vi "Visualizacion_NEW.vi"() -> ()   [LabVIEW 2021]
uses:
  <vilib>/Modbus/master/Modbus Master.lvclass
  <vilib>/Modbus/master/Create Master Instance (TCP).vi
panel:
  out "LEL":bool
  out "CO":bool
  out "O2":bool
  out "Contador Ciclos":sgl
  out "LEL":sgl
  out "CO":sgl
  out "O2":sgl
  in  "SP Temperatura (CC)":dbl=25.0 min=-42.0 max=55.0
  in  "SP HR (CC)":dbl=10.0
  out "DI Sim Bitron Param":bool
  out "Parameters":u16[](array[numeric])
  out "Error":bool
  out "Warning":bool
  out "MEAN (T)":sgl format="%0.2f"
  out "Peltiers enable":bool
  out "Program Status":bool
  out "SP (T)":sgl
  out "Segmento_temp":u16
  in  "?":T1(tab)
  in  "?":T2(tab)
  out "TEMPERATURA MEDIA":dynamicdata(graph)
  out "ALL TOGETHER":dynamicdata(graph)
  out "VALVULA 1  BOBINAS 1 Y 2":dynamicdata(graph)
  out "VALVULA 2 Y BOBINA 3 Y 4":dynamicdata(graph)
  out "VALVULA 3 Y BOBINA 5 Y 6":dynamicdata(graph)
  out "VALVULA 4 Y BOBINA 7 Y 8":dynamicdata(graph)
  out "O2/CO/LEL":dynamicdata(graph)
  out "Camara climatica":dynamicdata(graph)
  out "current time":timestamp
  out "W1.16":bool
  out "W1.15":bool
  out "W1.11":bool
  out "W1.10":bool
  out "W1.14":bool
  out "W1.13":bool
  out "W1.12":bool
  out "W1.1":bool
  out "W2":bool
  out "W3":bool
  out "W4":bool
  out "W1.2":bool
  out "W1.3":bool
  out "W1.6":bool
  out "W1.5":bool
  out "W1.4":bool
  out "W1.9":bool
  out "W1.8":bool
  out "W1.7":bool
  out "warnings table":T3(array[cluster]) {"Time Stamp" format="%<%.3X %x>T"}
  in  "Reset":bool
  out "Comunicacion Modbus":errorcluster
  in  "trigger bob frio (ºC)":dbl=-27.5 min=-40.0 max=80.0
  in  "Offset de ciclo.":dbl min=-40.0 max=80.0
  in  "Digital Input Bitron Simulation":bool
  in  "Pelt ºC/min":dbl=6.0
  in  "Cam ºC/min":dbl=100.0
  in  "Tiempo máximo de ciclo(min)":dbl=140.0
  in  "Setpoint corte frío(ºC)":dbl=-30.0 min=-42.0 max=80.0
  in  "Setpoint Frío(ºC)":dbl=-33.0 min=-42.0 max=80.0
  in  "Setpoint peltiers(ºC)":dbl=85.0 min=-42.0 max=80.0
  in  "Tiempo estabilidad de Frío(min)":dbl=15.0
  in  "Tiempo mínimo de ciclo(min)":dbl=70.0
  in  "Setpoint calor corte rampa(ºC)":dbl=51.0 min=-40.0 max=80.0
  in  "Tiempo ciclo (Bitron FSM Sim)":dbl=95.0
  in  "Setpoint calor cam":dbl=55.0 min=-40.0 max=80.0
  in  "Tiempo Ciclo 0 (min)":dbl=5.0
  in  "Save Parameters":bool
  out "Ventil 2":sgl
  out "Ventil 3":sgl format="%#.2g"
  out "Temp bob 1 (P)":sgl format="%#.2g"
  out "Temp bob 3 (P)":sgl
  out "Ventil 4":sgl
  out "Ventil 1":sgl format="%#.2g"
  out "Temp Bob 5 (P)":sgl format="%#.2g"
  in  "PWM 4(SP)":u16
  in  "PWM 3(SP) 2":u16
  in  "PWM 2(SP) 2":u16
  in  "PWM 1(SP) 2":u16
  in  "Test PWM (%)":bool
  in  "Conf PIDs":bool
  in  "TestPID 4(ºC)":u16
  in  "TestPID3(ºC)":u16
  in  "TestPID 2(ºC)":u16
  in  "TestPID 1(ºC)":u16
  out "Temp Man 2":sgl
  out "PWM 1(SP)":u16
  out "Temp Man 3":sgl format="%#.2g"
  out "Temp Man 1":sgl format="%#.2g"
  out "Temp Man 4":sgl
  out "PWM 2(SP)":u16
  out "PWM 3(SP)":u16
  out "PWM 4(SP)":u16
  out "Temp bob 7 (P)":sgl
  out "Temp bob 2 (Sh)":sgl
  out "Temp bob  4 (Sh)":sgl
  out "Temp bob 6 (Sh)":sgl format="%#.2g"
  out "Temp bob 8 (Sh)":sgl
  in  "Descarte Media Temps":u16 max=3 step=1
  in  "Enable PI 1":bool=TRUE
  in  "Enable PI 2":bool=TRUE
  in  "Enable PI 3":bool=TRUE
  in  "Enable PI 4":bool=TRUE
  in  "Test PID (ºC)":bool
  out "DISK":sgl(graph)
  out "RAM":sgl(graph)
  in  "Tiempo de guardado":u32=600
  out "data to be saved":dbl[][](array[numeric])
  out "Guardando en disco":bool
  out "array w/ subset deleted":dbl[][](array[numeric])
  out "size(s)":i32
  out "W to save":string[][](array[string])
  in  "Warning saved":bool
  in  "Tiempo/dato (s)":u32=1
  out "USO DE DISCO(%)":sgl
  out "USO DE RAM (%)":sgl
  out "DO H2 Lab":bool
  in  "Guardar datos":bool=TRUE
  out "senal_bitron":bool
  in  "Stop Ensayo":bool
  out "Coils write":bool[](array[boolean])
  out "Int values":u16[](array[numeric])
  out "SGL values":sgl[](array[numeric])
  out "coil values":bool[](array[boolean])
  out "ComunicacionCRIO":bool
  in  "run_program":bool
  out "Setpoint_temp_write":dbl
  out "Setpoint_hum_write":dbl
  out "Temperatura Camara":dbl
  out "Humedad relativa (HR)":dbl
  in  "Pause_Entrar_camara":bool
  in  "Pause":bool
  in  "stop":bool
  in  "Tab Control":T4(tab)
  out "T Man 4":dbl(slide) scale=-45.0..100.0
  out "T Man 3":dbl(slide) scale=-45.0..100.0
  out "T Man 2":dbl(slide) scale=-45.0..100.0
  out "T Man 1":dbl(slide) scale=-45.0..100.0
  out "T Bob 1":dbl(slide) scale=-40.0..95.0
  out "T Bob 3":dbl(slide) scale=-40.0..95.0
  out "T Bob 5":dbl(slide) scale=-40.0..100.0
  out "T bob 9":dbl(slide) scale=-40.0..95.0
  out "T bob 10":dbl(slide) scale=-40.0..95.0
  out "T bob 11":dbl(slide) scale=-40.0..95.0
  out "T Bob 7":dbl(slide) scale=-40.0..95.0
  out "T bob 12":dbl(slide) scale=-45.0..95.0
  out "T bob 8":dbl(slide) scale=-45.0..95.0
  out "T bob 7":dbl(slide) scale=-45.0..95.0
  out "T bob 6":dbl(slide) scale=-45.0..95.0
  out "Ventil 5":dbl(slide) scale=-45.0..95.0
  # "Control Programa Principal"
  # "Control Manual CC"
  # "%"
  # "ºC"
  # "Cámara climática"
  # "ºC"
  # "ºC"
  # "%"
  # "%"
  # "Simulación señal Bitron"
  # "ºC"
  # "HR"
  # "TempCC"
  # "SP_HR"
  # "SP_TempCC"
  # "Mean T"
  # "Warnings y Errores"
  # "Warning Valvulas"
  # "Warning Bobinas"
  # "Parametros y configuracion para la curva de ciclado"
  # "ºC"
  # "VALVE 4"
  # "ºC"
  # "ºC"
  # "Fan Right"
  # "%"
  # "ºC"
  # "ºC"
  # "VALVE 3"
  # "ºC"
  # "ºC"
  # "%"
  # "Fan Mid-Right"
  # "ºC"
  # "ºC"
  # "VALVE 2"
  # "ºC"
  # "ºC"
  # "%"
  # "Fan Mid-Left"
  # "ºC"
  # "ºC"
  # "VALVE 1"
  # "ºC"
  # "ºC"
  # "%"
  # "Fan Left"
  # "ºC"
  # "ºC"
  # "1 Dato\n----------------"
  # "Frecuencia de guardado:"
  # "s"
  # "s"
  # "T Manifolds:"
  # "1                              2                                 3                                  4"
  # "T Bobinas:"
  # "1               2               3               4               5                 6               7               8"
  # "V1"
  # "V2"
  # "V3"
  # "V4"
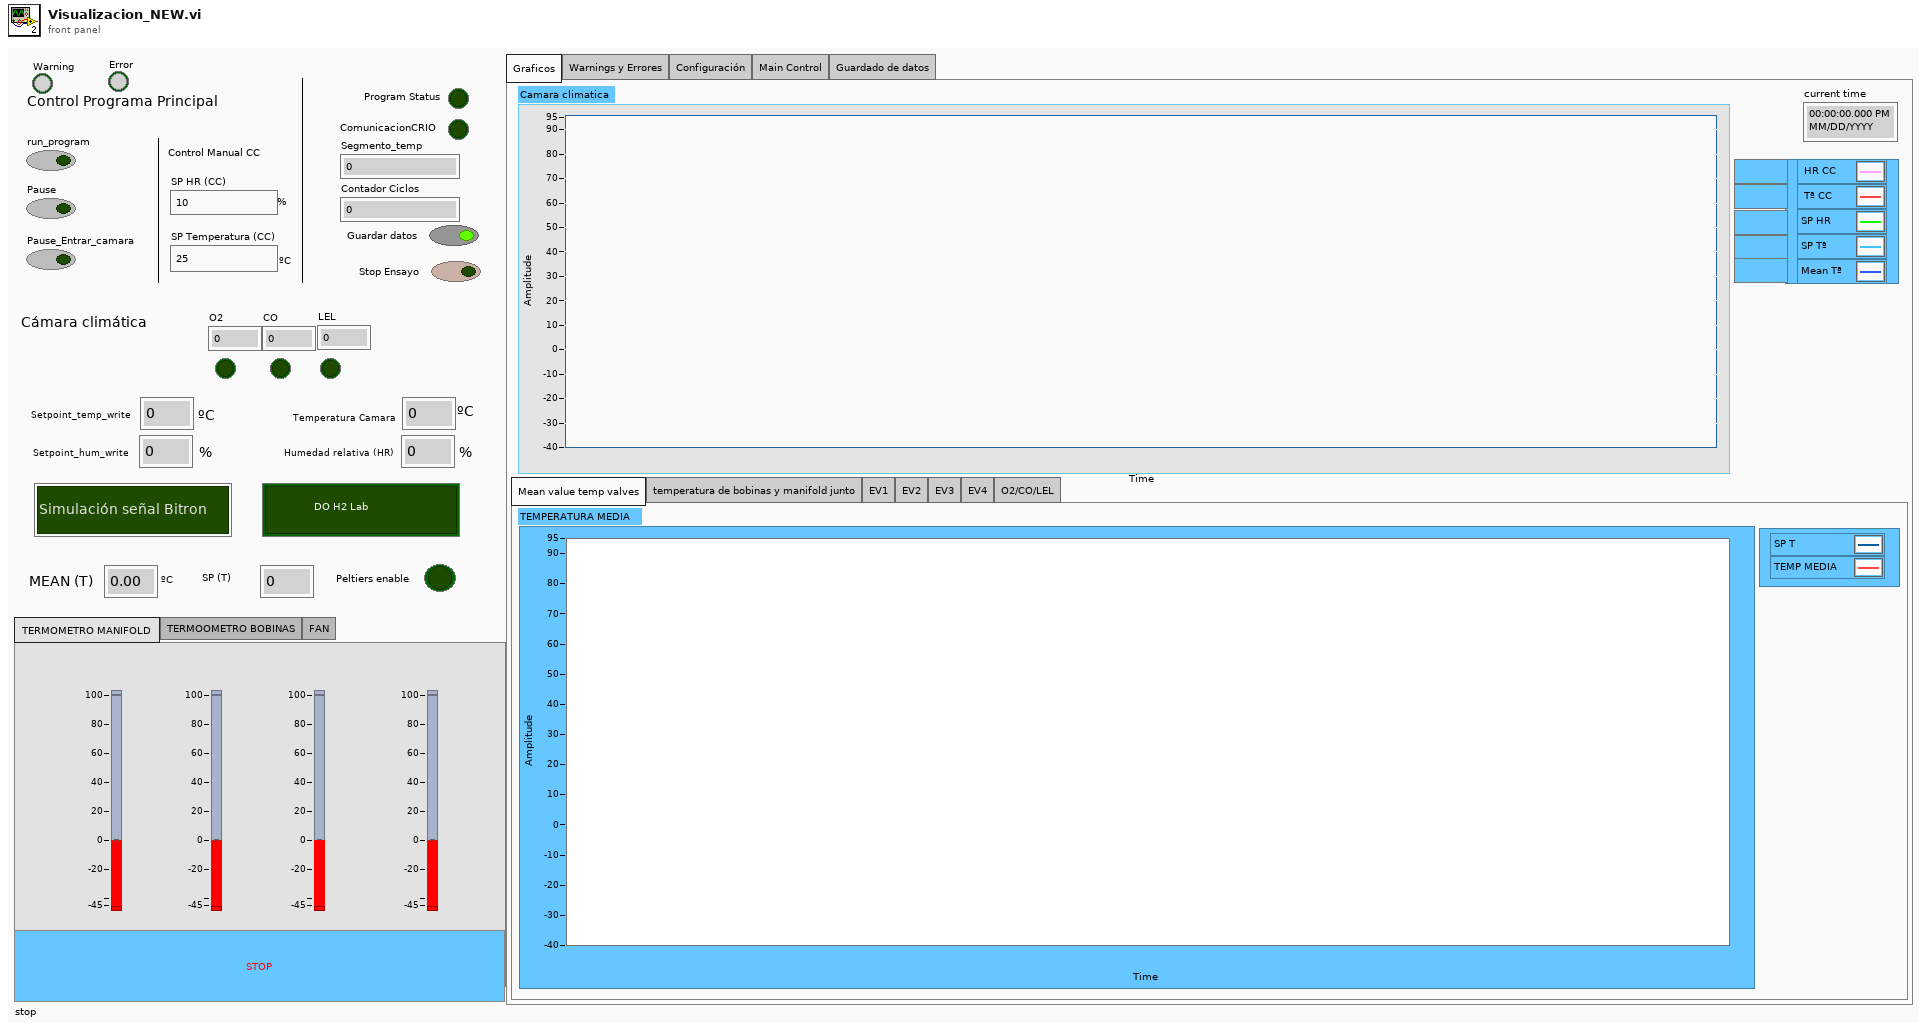
[diagram p1: front panel]
types:
  T1 = enum32{"Graficos", "Warnings y Errores", "Configuración", "Main Control", "Guardado de datos"}
  T2 = enum32{"Mean value temp valves", "temperatura de bobinas y manifold junto", "EV1", "EV2", "EV3", "EV4", "O2/CO/LEL"}
  T3 = cluster{"Time Stamp":timestamp, "Descripcion":string, "Numeric":i32}[]
  T4 = enum32{"TERMOMETRO MANIFOLD ", "TERMOOMETRO BOBINAS", "FAN"}
  T5 = enum8{"Enabled", "Disabled", "Disabled and Grayed Out"}
  T6 = enum16{"open", "open or create", "create or replace", "create", "open (read-only)"}
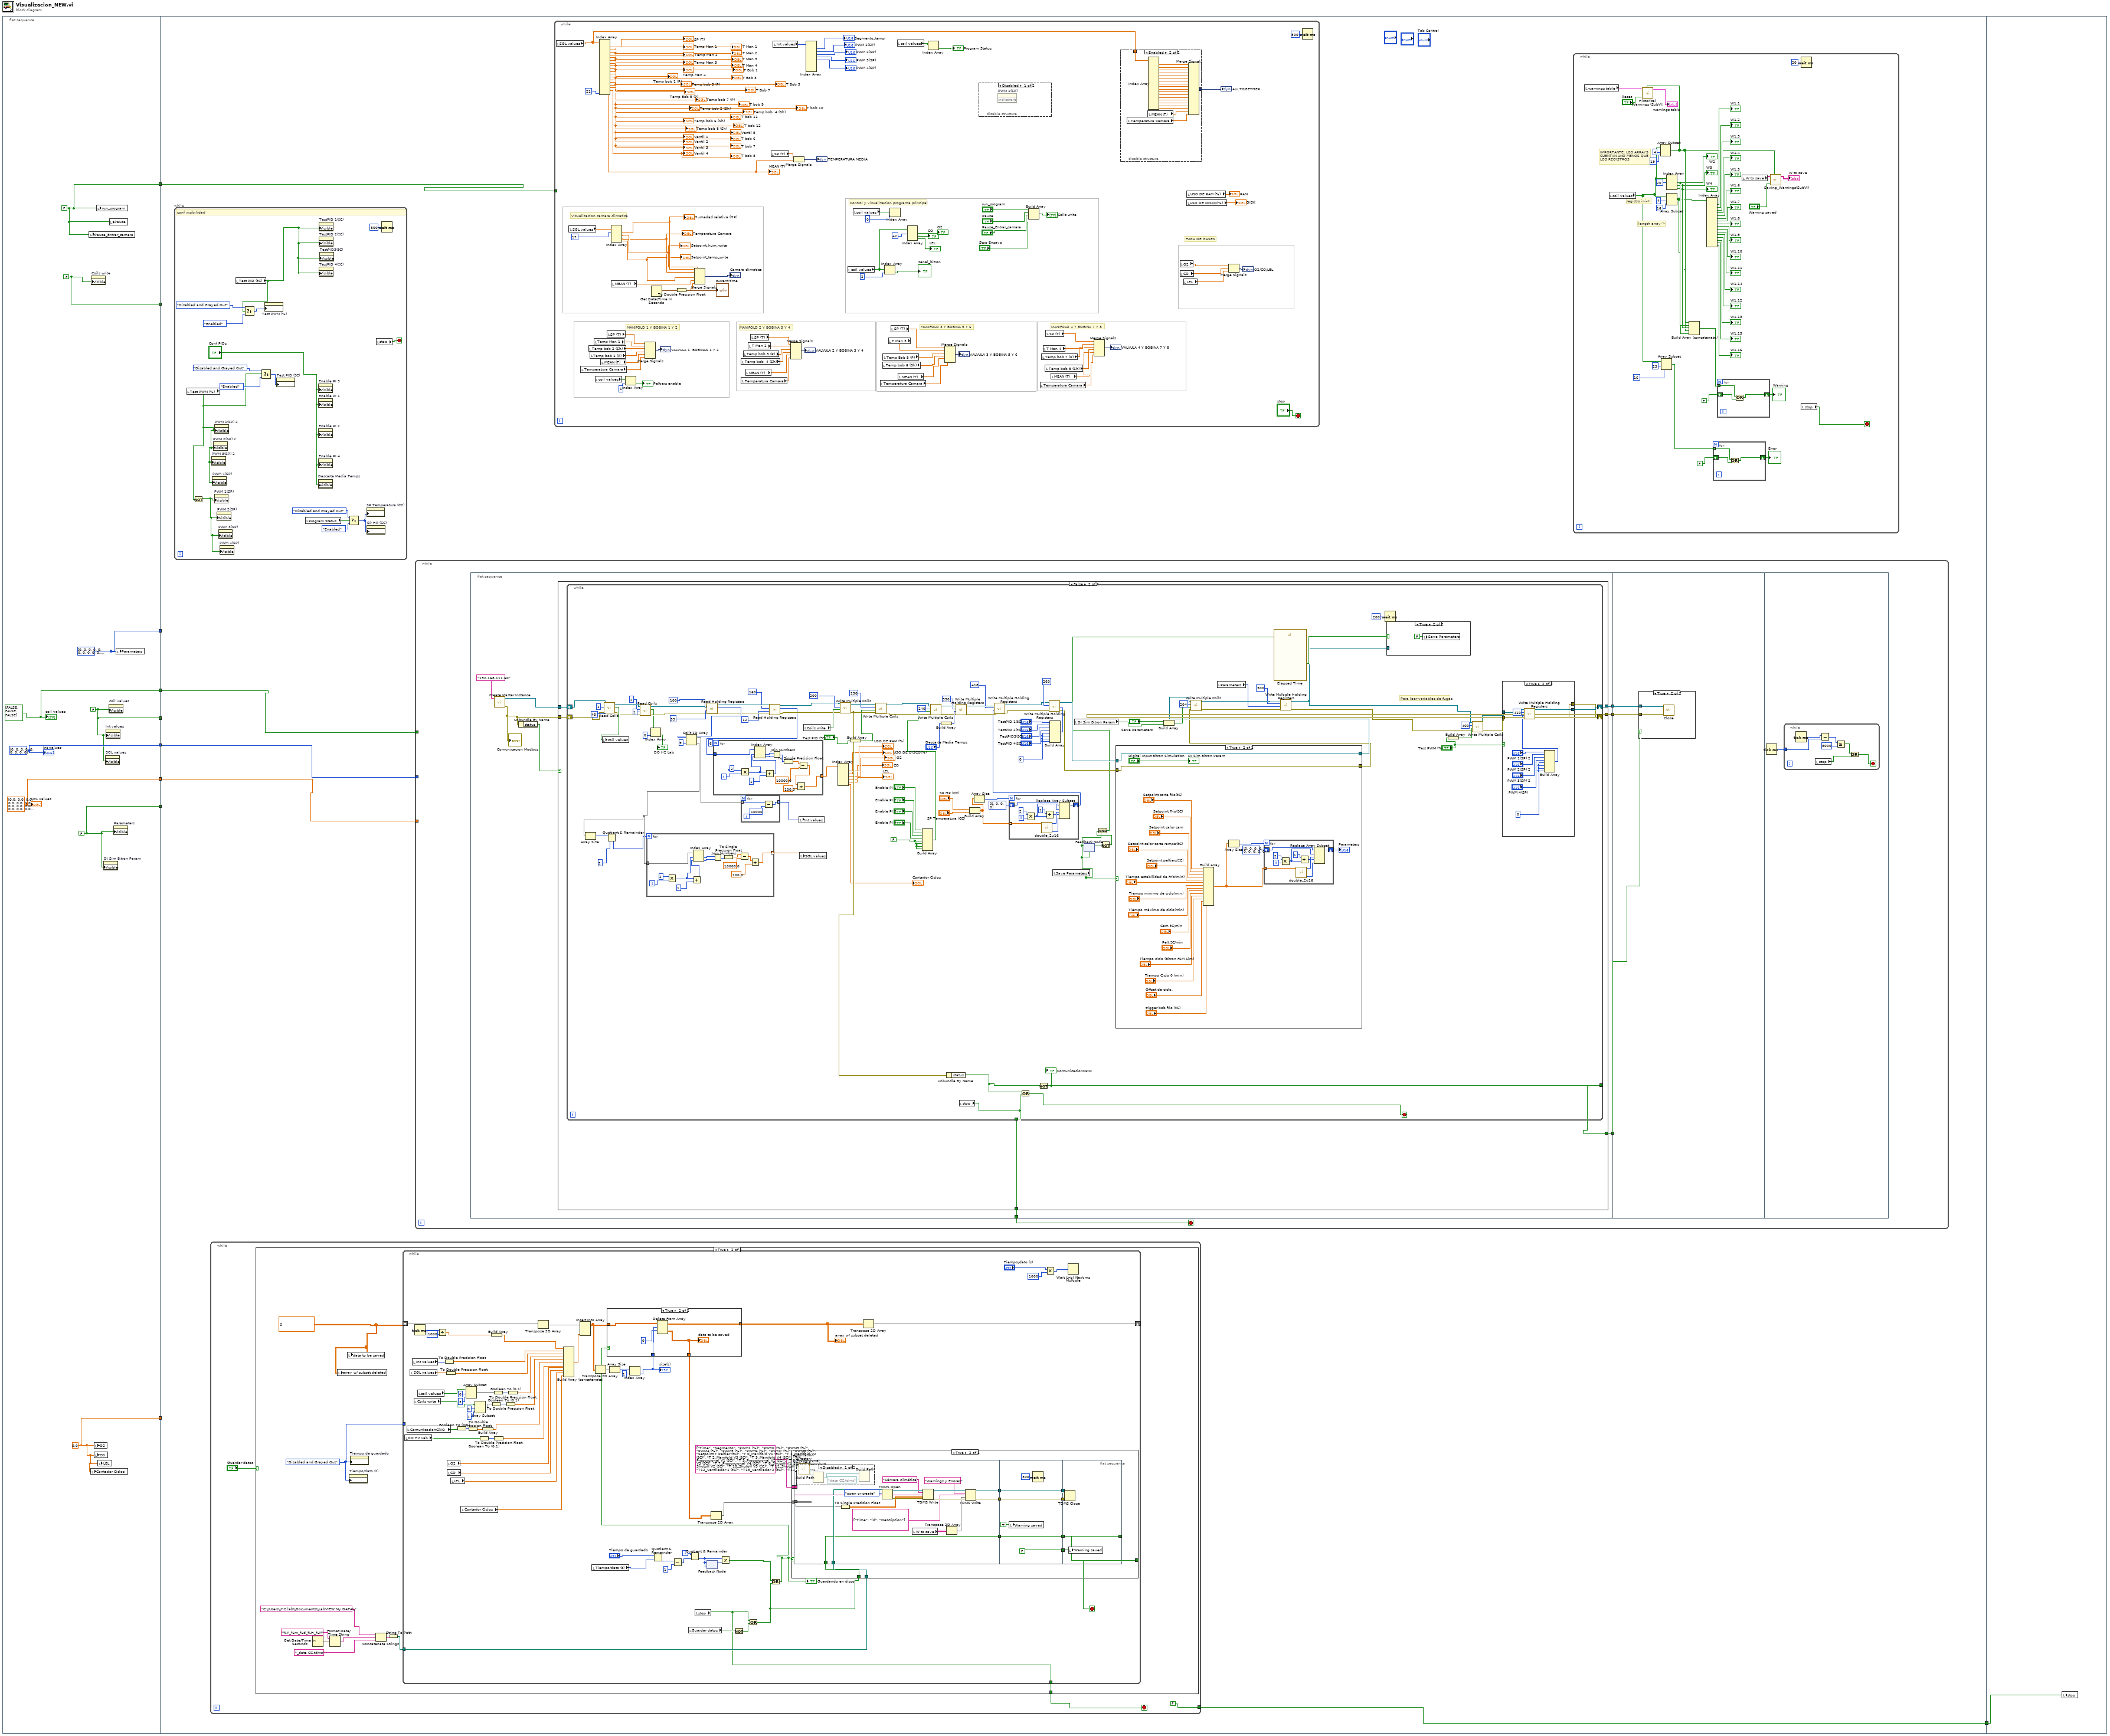
[diagram p0: block diagram]
diagram:
  n1 = flat-sequence {
    tunnel: [w19] -> w10
    tunnel: [w18] -> w9
    tunnel: [w17] -> w8
    tunnel: [w16] -> w7
    tunnel: [w14] -> w5
    tunnel: [w15] -> w4
    tunnel: [w13] -> w3
    tunnel: [w12] -> w2
    tunnel: [w11] -> w1
    tunnel: w10 -> [w24]
    tunnel: w9 -> [w23]
    tunnel: w8 -> [w22]
    tunnel: w7 -> [w21]
    tunnel: [w20] -> w6
    tunnel: w5 -> [_]
    tunnel: w4 -> [_]
    tunnel: w3 -> [_]
    tunnel: w2 -> [_]
    tunnel: w1 -> [_]
    tunnel: w6 -> [w583]
    frame #0 {
      w11 = sgl 0.0 ("O2")
      w12 = u16[] [0, 0, 0, 0, 0, 0, 0, 0, 0, 0, 0, 0, 0, 0, 0, 0, 0, 0, 0, 0, 0, 0] ("Parameters")
      w13 = FALSE ("Visible")
      w15 = FALSE ("Visible")
      w14 = FALSE ("Visible")
      w17 = sgl[] [0.0, 0.0, 0.0, 0.0, 0.0, 0.0, 0.0, 0.0, 0.0, 0.0, 0.0, 0.0, 0.0, 0.0, 0.0, 0.0, 0.0, 0.0, 0.0, 0.0, 0.0, 0.0] ("SGL values")
      w18 = u16[] [0, 0, 0, 0, 0, 0, 0, 0, 0] ("Int values")
      w16 = FALSE ("run_program")
      w19 = bool[] [FALSE, FALSE, FALSE] ("coil values")
      n2 = local write "Pause_Entrar_camara"(w16) -> ()
      n3 = local write "Contador Ciclos"(w11) -> ()
      n4 = property on="Coils write" class="Arr (strict)"("Visible"=w15) -> ()  [unwired: 2 in, 2 out]
      n5 = local write "O2"(w11) -> ()
      n6 = local write "CO"(w11) -> ()
      n7 = local write "run_program"(w16) -> ()
      n8 = local write "LEL"(w11) -> ()
      n9 = property on="DI Sim Bitron Param" class="Bool (strict)"("Visible"=w13) -> ()  [unwired: 2 in, 2 out]
      n10 = property on="SGL values" class="Arr (strict)"("Visible"=w14) -> ()  [unwired: 2 in, 2 out]
      n11 = property on="Int values" class="Arr (strict)"("Visible"=w14) -> ()  [unwired: 2 in, 2 out]
      n12 = property on="coil values" class="Arr (strict)"("Visible"=w14) -> ()  [unwired: 2 in, 2 out]
      n13 = local write "Pause"(w16) -> ()
      n14 = property on="Parameters" class="Arr (strict)"("Visible"=w13) -> ()  [unwired: 2 in, 2 out]
      n15 = local write "Parameters"(w12) -> ()
      "coil values" <- w19
      "Int values" <- w18
      "SGL values" <- w17
    }
    frame #1 {
      n16 = while {
        stop <- w40 stop-if-true
        # "conf visibilidad"
        n17 = local read "Test PWM (%)"() -> (w29:bool)
        n18 = Not(x=w29) -> (.not. x?=w37:bool)
        n19 = property on="PWM 3(SP) 2" class="DigNum (strict)"("Visible"=w29) -> ()  [unwired: 2 in, 2 out]
        n20 = property on="PWM 4(SP)" class="DigNum (strict)"("Visible"=w29) -> ()  [unwired: 2 in, 2 out]
        n21 = property on="PWM 2(SP) 2" class="DigNum (strict)"("Visible"=w29) -> ()  [unwired: 2 in, 2 out]
        n22 = property on="PWM 1(SP)" class="DigNum (strict)"("Visible"=w37) -> ()  [unwired: 2 in, 2 out]
        n23 = property on="PWM 1(SP) 2" class="DigNum (strict)"("Visible"=w29) -> ()  [unwired: 2 in, 2 out]
        n24 = property on="PWM 2(SP)" class="DigNum (strict)"("Visible"=w37) -> ()  [unwired: 2 in, 2 out]
        n25 = property on="PWM 3(SP)" class="DigNum (strict)"("Visible"=w37) -> ()  [unwired: 2 in, 2 out]
        n26 = property on="PWM 4(SP)" class="DigNum (strict)"("Visible"=w37) -> ()  [unwired: 2 in, 2 out]
        n27 = local read "Test PID (ºC)"() -> (w33:bool)
        n28 = Select(t=T5."Disabled and Grayed Out" ("Disabled"), s=w33, f=T5."Enabled" ("Disabled")) -> (s? t:f=w34:T5)
        n29 = Select(t=T5."Disabled and Grayed Out" ("Disabled"), s=w29, f=T5."Enabled" ("Disabled")) -> (s? t:f=w30:T5)
        n30 = property on="Test PWM (%)" class="Bool (strict)"("DisabledEnum"=w34) -> ()  [unwired: 2 in, 2 out]
        n31 = property on="Test PID (ºC)" class="Bool (strict)"("DisabledEnum"=w30) -> ()  [unwired: 2 in, 2 out]
        n32 = local read "Program Status"() -> (w28:bool)
        n33 = property on="Descarte Media Temps" class="DigNum (strict)"("Visible"="Conf PIDs") -> ()  [unwired: 2 in, 2 out]
        n34 = property on="Enable PI 3" class="Bool (strict)"("Visible"="Conf PIDs") -> ()  [unwired: 2 in, 2 out]
        n35 = property on="Enable PI 1" class="Bool (strict)"("Visible"="Conf PIDs") -> ()  [unwired: 2 in, 2 out]
        n36 = property on="Enable PI 2" class="Bool (strict)"("Visible"="Conf PIDs") -> ()  [unwired: 2 in, 2 out]
        n37 = property on="Enable PI 4" class="Bool (strict)"("Visible"="Conf PIDs") -> ()  [unwired: 2 in, 2 out]
        n38 = property on="TestPID 1(ºC)" class="DigNum (strict)"("Visible"=w33) -> ()  [unwired: 2 in, 2 out]
        n39 = property on="TestPID 2(ºC)" class="DigNum (strict)"("Visible"=w33) -> ()  [unwired: 2 in, 2 out]
        n40 = property on="TestPID 4(ºC)" class="DigNum (strict)"("Visible"=w33) -> ()  [unwired: 2 in, 2 out]
        n41 = property on="TestPID3(ºC)" class="DigNum (strict)"("Visible"=w33) -> ()  [unwired: 2 in, 2 out]
        n42 = Select(t=T5."Disabled and Grayed Out" ("Disabled"), s=w28, f=T5."Enabled" ("Disabled")) -> (s? t:f=w25:T5)
        n43 = property on="SP Temperatura (CC)" class="DigNum (strict)"("DisabledEnum"=w25) -> ()  [unwired: 2 in, 2 out]
        n44 = property on="SP HR (CC)" class="DigNum (strict)"("DisabledEnum"=w25) -> ()  [unwired: 2 in, 2 out]
        n45 = local read "stop"() -> (w40:bool)
        n46 = Wait (ms)(milliseconds to wait=u32 500) -> ()  [unwired: 1 out]
      }
      n47 = while {
        tunnel: [FALSE ("stop Control General")] -> w20
        stop <- w91 stop-if-true
        n48 = case shown="True" "Guardar datos" {
          tunnel: [w94 w97] -> w91
          frame False {
            w93 = T5."Enabled" ("Disabled")
            n49 = property on="Tiempo/dato (s)" class="DigNum (strict)"("DisabledEnum"=w93) -> ()  [unwired: 2 in, 2 out]
            n50 = property on="Tiempo de guardado" class="DigNum (strict)"("DisabledEnum"=w93) -> ()  [unwired: 2 in, 2 out]
            n51 = local read "stop"() -> (w94:bool)
            n52 = Wait Until Next ms Multiple(millisecond multiple=u32 1000 ("milliseconds to wait")) -> ()  [unwired: 1 out]
          }
          frame True {
            w96 = T5."Disabled and Grayed Out" ("Disabled")
            w105 = dbl[][] []
            n53 = Get Date/Time In Seconds() -> (seconds since 1Jan1904=w104:timestamp)
            n54 = Format Date/Time String(time format string (%c)="%Y_%m_%d_%H_%M", seconds (now)=w104) -> (date/time string=w101:string)  [unwired: 1 in]
            n55 = local write "array w/ subset deleted"(w105) -> ()
            n56 = local write "data to be saved"(w105) -> ()
            n57 = property on="Tiempo/dato (s)" class="DigNum (strict)"("DisabledEnum"=w96) -> ()  [unwired: 2 in, 2 out]
            n58 = property on="Tiempo de guardado" class="DigNum (strict)"("DisabledEnum"=w96) -> ()  [unwired: 2 in, 2 out]
            n59 = Concatenate Strings("C:\\Users\\H2.lab\\Documents\\LabVIEW My DATA\\" ("string"), w101, "_data CC.tdms" ("string")) -> (w102:string)
            n60 = String To Path(string=w102) -> (path=w99:path)
            n61 = while {
              shift-right: [w160] -> _
              shift-left: w105 -> [w163]
              tunnel: w99 -> [w153]
              tunnel: [w131] -> w97
              tunnel: w96 -> [_]
              i -> [w167]
              stop <- w135 stop-if-true
              n62 = local read "DO H2 Lab"() -> (w129:bool)
              n63 = local read "ComunicacionCRIO"() -> (w137:bool)
              n64 = local read "SGL values"() -> (w151:sgl[])
              n65 = local read "Int values"() -> (w152:u16[])
              n66 = local read "Coils write"() -> (w123:bool[])
              n67 = Tick Count (ms)() -> (millisecond timer value=w155:u32)
              n68 = local read "coil values"() -> (w127:bool[])
              n69 = Divide(x=w155, y=u32 1000) -> (x/y=w148:dbl)
              n70 = To Double Precision Float(number=w152) -> (double precision float=w150:dbl[])
              n71 = To Double Precision Float(number=w151) -> (double precision float=w149:dbl[])
              n72 = local read "O2"() -> (w110:sgl)
              n73 = local read "CO"() -> (w109:sgl)
              n74 = local read "LEL"() -> (w108:sgl)
              n75 = Boolean To (0,1)(Boolean=w137) -> (0, 1=w144:i16)
              n76 = local read "Contador Ciclos"() -> (w107:sgl)
              n77 = Array Subset(array=w127, index=0, length=3) -> (w126:bool[])
              n78 = To Double Precision Float(number=w144) -> (double precision float=w143:dbl)
              n79 = Array Subset(array=w123, index=0, length=4) -> (w120:bool[])
              n80 = Boolean To (0,1)(Boolean=w129) -> (0, 1=w130:i16)
              n81 = Build Array(w143) -> (w140:dbl[])
              n82 = Boolean To (0,1)(Boolean=w120) -> (0, 1=w139:i16[])
              n83 = Build Array(w148) -> (w147:dbl[])
              n84 = Boolean To (0,1)(Boolean=w126) -> (0, 1=w146:i16[])
              n85 = To Double Precision Float(number=w130) -> (double precision float=w128:dbl)
              n86 = To Double Precision Float(number=w139) -> (double precision float=w138:dbl[])
              n87 = To Double Precision Float(number=w146) -> (double precision float=w145:dbl[])
              n88 = Transpose 2D Array(2D array=w163) -> (transposed array=w162:dbl[][])
              n89 = Build Array (concatenate)(w147, w150, w149, w145, w138, w140, w128, w110, w109, w108, w107) -> (w168:dbl[])
              n90 = Insert Into Array(array=w162, new element=w168) -> (w165:dbl[][])  [unwired: 2 in]
              n91 = local read "Tiempo/dato (s)"() -> (w115:u32)
              n92 = Transpose 2D Array(2D array=w165) -> (transposed array=w159:dbl[][])
              n93 = Array Size(array=w159) -> (size(s)=w158:i32[])
              n94 = Index Array(array=w158, index=1) -> (element=w157:i32)
              "size(s)" <- w157
              n95 = Quotient & Remainder(x="Tiempo de guardado", y=w115) -> (floor(x/y)=w114:u32)  [unwired: 1 out]
              n96 = Subtract(x=w114, y=u32 1) -> (x-y=w113:u32)
              n97 = local read "Guardar datos"() -> (w134:bool)
              n98 = Quotient & Remainder(x=w167, y=w113) -> (floor(x/y)=w164:u32)  [unwired: 1 out]
              n99 = local read "stop"() -> (w131:bool)
              n100 = feedback-in #1(w164) -> ()
              n101 = feedback #1(w164) -> (w166:u32)
              n102 = Not Equal?(x=w164, y=w166) -> (x != y?=w136:bool)
              n103 = Not(x=w134) -> (.not. x?=w133:bool)
              n104 = Or(x=w131, y=w133) -> (x .or. y?=w132:bool)
              n105 = Or(x=w136, y=w132) -> (x .or. y?=w142:bool)
              "Guardando en disco" <- w142
              n106 = case shown="True" w142 {
                tunnel: w165 -> [w170 w173]
                tunnel: [w170 w175] -> w161
                tunnel: w157 -> [_ w172]
                tunnel: [dbl[][] [] w171] -> w141
                frame False {
                }
                frame True {
                  n107 = Delete From Array(array=w173, length=w172, index (row)=0) -> (deleted portion=w171:dbl[][], array with subset deleted=w175:dbl[][])  [unwired: 1 in]
                  "data to be saved" <- w171
                }
              }
              "array w/ subset deleted" <- w161
              n108 = Transpose 2D Array(2D array=w141) -> (transposed array=w111:dbl[][])
              n109 = case shown="True" w142 {
                tunnel: string[] ["Time", "Segmento", "PWM1 (%)", "PWM2 (%)", "PWM3 (%)", "PWM4 (%)", "PWM5 (%)", "PWM6 (%)", "PWM7 (%)", "PWM8 (%)", "Setpoint T Peltier (ºC)", "T 0_Manifold V1 (ºC)", "T 1_Manifold V2 (ºC)", "T 2_Manifold V3 (ºC)", "T 3_Manifold V4 (ºC)", "T 4_Proporcional V1 (ºC)", "T 5_Proporcional V2 (ºC)", "T 6_Proporcional V3 (ºC)", "T 7_Proporcional V4 (ºC)", "T 8_Shutoff V1 (ºC)", "T 9_Shutoff V2 (ºC)", "T 10_Shutoff V3 (ºC)", "T 11_Shutoff V4 (ºC)", "T12_Ventilador 1 (ºC)", "T13_Ventilador 2 (ºC)", "T14_ Ambiente panel (ºC)", "T15_Panel (ºC)", "HR RD CC (%)", "SP HR WR CC (%)", "T RD CC (ºC)", "SP T WR CC (ºC)", "Mean TBobs (ºC)", "Program Status", "Enable PI", "Entrada Bitron", "Run Program", "Pause", "Pause Entrar", "Stop control general", "Comunicacion con PC", "DO H2 Lab", "O2 (%)", "CO (ppm)", "LEL (%)", "Numero de ciclo"] -> [_ w188]
                tunnel: w111 -> [_ w187]
                tunnel: w153 -> [_ w186]
                tunnel: w132 -> [_ w185]
                tunnel: [FALSE ("STOP ALL") w184] -> w135
                frame False {
                }
                frame True {
                  n110 = flat-sequence {
                    tunnel: w188 -> [w201]
                    tunnel: w187 -> [w190]
                    tunnel: w186 -> [w200]
                    tunnel: w185 -> [w199]
                    tunnel: [w199] -> w183
                    tunnel: [w194] -> w180
                    tunnel: [w193] -> w178
                    tunnel: w183 -> [w214]
                    tunnel: [w214] -> w182
                    tunnel: [w213] -> w181
                    tunnel: w180 -> [w213]
                    tunnel: [w212] -> w179
                    tunnel: w178 -> [w212]
                    tunnel: [FALSE ("Warning saved")] -> w177
                    tunnel: [w218] -> w184
                    tunnel: w182 -> [w218]
                    tunnel: w181 -> [w217]
                    tunnel: w179 -> [w216]
                    tunnel: w177 -> [w215]
                    frame #0 {
                      n111 = disable-structure shown="Disabled" {
                        frame Disabled {
                          n112 = call <vilib>:"Application Directory.vi"() -> ("Application Directory"=w207:path)
                          n113 = Build Path(base path=w207) -> (appended path=w206:path)  [unwired: 1 in]
                          n114 = Build Path(base path=w206, name or relative path=path "data CC.tdms") -> ()  [unwired: 1 out]
                        }
                        frame Enabled {
                        }
                      }
                      n115 = To Single Precision Float(number=w190) -> (single precision float=w189:sgl[][])
                      n116 = TDMS Open(10:T6."open or create" ("operation (0:open)"), 11:w200) -> (0:w203:errorcluster, 3:w204:refnum<k34>)  [unwired: 5 in]
                      n117 = local read "W to save"() -> (w191:string[][])
                      n118 = TDMS Write(0:w204, 5:"Cámara climática" ("group name in (Untitled)"), 7:w201, 9:w189, 11:w203) -> (4:w198:refnum<k34>, 15:w197:errorcluster)  [unwired: 1 in, 2 out]
                      n119 = Transpose 2D Array(2D array=w191) -> (transposed array=w192:string[][])
                      n120 = TDMS Write(0:w198, 5:"Warnings y Errores" ("group name in (Untitled)"), 7:string[] ["Time", "id", "Description"] ("channel name(s) in (Untitled)"), 9:w192, 11:w197) -> (4:w193:refnum<k34>, 15:w194:errorcluster)  [unwired: 1 in, 2 out]
                    }
                    frame #1 {
                      n121 = local write "Warning saved"(TRUE ("Warning saved")) -> ()
                      n122 = Wait (ms)(milliseconds to wait=u32 300) -> ()  [unwired: 1 out]
                    }
                    frame #2 {
                      n123 = TDMS Close(8:w217, 11:w216) -> ()  [unwired: 2 out]
                      n124 = local write "Warning saved"(w215) -> ()